vi "UHR-Fleezers Control (host) - 10.0.vi"() -> ()   [LabVIEW 2009] (continued)
              }
            }
          }
        }
        n1053 = node-c288(w4126) -> ()  [unwired: 1 out]
      }
      n1054 = node-c288(w4110) -> ()  [unwired: 1 out]
      n1055 = call "DMR_CloseDevice.vi"("driver handle IN"=w4115) -> ()  [unwired: 1 in, 4 out]
    }
    frame #4 {
      n1056 = call "DMR_Close.vi"() -> ()  [unwired: 1 out]
    }
  }
  n1057 = disable-structure shown="Disabled" {
    disable-tunnel: [w4249 _] -> w213
    disable-tunnel: w14 -> [w4248 _]
    frame #0 {
      n1058 = node-c288() -> (w4251:T22)  [unwired: 4 out]
      n1059 = timed-loop "Rough control of MCL mirror stage (debugging)" {
        tunnel: w4248 -> [w4254]
        tunnel: [w4253] -> w4249
        timing: w4251 -> [_]
        timing-out: [_] -> w4250
        stop <- w4253 stop-if-true
        n1060 = node-c288() -> ()  [unwired: 2 out]
        n1061 = case shown="1" "MCL Mode" {
          tunnel: w4254 -> [_ w4257 w4359]
          frame #0 {
          }
          frame #1 {
            n1062 = node-c288() -> (w4259:T22)  [unwired: 4 out]
            n1063 = timed-loop "Oscillate MCL mirror" {
              timing: w4259 -> [_]
              timing-out: [_] -> w4258
              tunnel: w4257 -> [w4298]
              i -> [w4297]
              stop <- w4260 stop-if-true
              n1064 = node-c288() -> (w4296:i64)  [unwired: 1 out]
              n1065 = Multiply(x="AO1", y=32767.0) -> (x*y=w4292:dbl)
              n1066 = Multiply(x="AO2", y=32767.0) -> (x*y=w4287:dbl)
              n1067 = Divide(x=w4292, y=10.0) -> (x/y=w4293:dbl)
              n1068 = Divide(x=w4287, y=10.0) -> (x/y=w4288:dbl)
              n1069 = To Word Integer(number=w4293) -> (16bit integer=w4285:i16)
              n1070 = To Word Integer(number=w4288) -> (16bit integer=w4284:i16)
              n1071 = Divide(x=w4296, y=i64 1000) -> (x/y=w4267:dbl)
              n1072 = Multiply(x=w4267, y=w4297) -> (x*y=w4278:dbl)
              n1073 = Multiply(x="Osc. freq. (Hz) 2", y=6.283185307179586) -> (x*y=w4279:dbl)
              n1074 = Multiply(x=w4279, y=w4278) -> (x*y=w4277:dbl)
              n1075 = Sine(x=w4277) -> (sin(x)=w4276:dbl)
              n1076 = Multiply(x=w4276, y="Osc. amp. (V)") -> (x*y=w4274:dbl)
              n1077 = Add(x=w4274, y="Osc. center (V)") -> (x+y=w4272:dbl)
              n1078 = Divide(x=w4272, y=10.0) -> (x/y=w4270:dbl)
              n1079 = Multiply(x=w4270, y=32767.0) -> (x*y=w4265:dbl)
              n1080 = Select(t=w4265, s="Scan axis", f=w4285) -> (s? t:f=w4283:dbl)
              n1081 = Select(t=w4284, s="Scan axis", f=w4265) -> (s? t:f=w4282:dbl)
              n1082 = local read "MCL Mode"() -> (w4264:u16)
              n1083 = Not Equal?(x=w4264, y=u16 1) -> (x != y?=w4261:bool)
              n1084 = local read "Stop All"() -> (w4262:bool)
              n1085 = xnode "Read/Write Control"("FPGA VI Reference In"=w4298, "AO1"=w4283, "AO2"=w4282) -> ()  [unwired: 1 in, 2 out]
              n1086 = Compound Arithmetic op=OR(w4262, w4261) -> (w4260:bool)
              n1087 = node-c288() -> ()  [unwired: 2 out]
            }
            n1088 = node-c288(w4258) -> ()  [unwired: 1 out]
          }
          frame #2 {
            n1089 = case shown="True" "Start Scan" {
              tunnel: w4359 -> [_ w4371]
              frame #0 {
              }
              frame #1 {
                n1090 = Subtract(x="End (V)", y="Begin (V)") -> (x-y=w4367:dbl)
                n1091 = Decrement(x="N Points") -> (x-1=w4366:dbl)
                n1092 = Divide(x=w4367, y=w4366) -> (x/y=w4364:dbl)
                n1093 = for {
                  N: "N Points" -> [_]
                  tunnel: "Begin (V)" -> [w4384]
                  tunnel: w4371 -> [w4376]
                  tunnel: [w4375] -> w4370 mode=indexing
                  tunnel: w4364 -> [w4374]
                  tunnel: [w4372] -> w4363 mode=indexing
                  i -> [w4383]
                  n1094 = Multiply(x=w4374, y=w4383) -> (x*y=w4382:dbl)
                  n1095 = Add(x=w4384, y=w4382) -> (x+y=w4379:dbl)
                  n1096 = local read "Scan axis"() -> (w4373:bool)
                  n1097 = local read "AO1"() -> (w4381:dbl)
                  n1098 = local read "AO2"() -> (w4380:dbl)
                  n1099 = Select(t=w4379, s=w4373, f=w4381) -> (s? t:f=w4378:dbl)
                  n1100 = Select(t=w4380, s=w4373, f=w4379) -> (s? t:f=w4377:dbl)
                  n1101 = flat-sequence {
                    tunnel: w4378 -> [w4388]
                    tunnel: w4377 -> [w4387]
                    tunnel: w4376 -> [w4385]
                    tunnel: [w4453] -> w4375
                    tunnel: [w4452] -> w4372
                    frame #0 {
                      w4391 = 10.0 ("y")
                      w4386 = 32767.0 ("y")
                      n1102 = Multiply(x=w4388, y=w4386) -> (x*y=w4394:dbl)
                      n1103 = Multiply(x=w4387, y=w4386) -> (x*y=w4392:dbl)
                      n1104 = Divide(x=w4394, y=w4391) -> (x/y=w4395:dbl)
                      n1105 = Divide(x=w4392, y=w4391) -> (x/y=w4393:dbl)
                      n1106 = To Word Integer(number=w4395) -> (16bit integer=w4389:i16)
                      n1107 = To Word Integer(number=w4393) -> (16bit integer=w4390:i16)
                      n1108 = xnode "Read/Write Control"("FPGA VI Reference In"=w4385, "AO1"=w4389, "AO2"=w4390) -> ()  [unwired: 1 in, 2 out]
                    }
                    frame #1 {
                      n1109 = Wait (ms)(milliseconds to wait="DAQ Delay (ms)") -> ()  [unwired: 1 out]
                    }
                    frame #2 {
                      n1110 = local read "Slow mean"() -> (w4453:dbl)
                      n1111 = local read "Sigma"() -> (w4452:dbl)
                    }
                  }
                }
                n1112 = Bundle("Begin (V)"="Begin (V)", w4364, w4370) -> (→"MCL Scan":cluster{"Begin (V)":dbl, dbl, dbl[]})  [unwired: 1 out]
                n1113 = Bundle("Begin (V)"="Begin (V)", w4364, w4363) -> (→"MCL Scan 2":cluster{"Begin (V)":dbl, dbl, dbl[]})  [unwired: 1 out]
              }
            }
          }
        }
        n1114 = local read "Stop All"() -> (w4253:bool)
        n1115 = node-c288() -> ()  [unwired: 2 out]
      }
      n1116 = node-c288(w4250) -> ()  [unwired: 1 out]
    }
    frame #1 {
    }
  }
  n1117 = timed-loop "Control parameters (event loop)" {
    tunnel: w14 -> [w4460]
    shift-right: [w4459] -> _
    shift-left: errorcluster {"status"=FALSE, "code"=0, "source"=""} ("error out") -> [w4458]
    tunnel: [w4457] -> w211
    timing: w52 -> [_]
    timing-out: [_] -> w51
    tunnel: w22 -> [w4456]
    stop <- w4457 stop-if-true
    n1118 = node-c288() -> ()  [unwired: 2 out]
    n1119 = event shown="[50] \"Set SP to Reading\": Value Change" {
      selector: _ -> [_ _ _ _ _ _ _ _ _ _ _ _ _ _ _ _ _ _ _ _ _ _ _ _ _ _ _ _ _ _ _ _ _ _ _ _ _ _ _ _ _ _ _ _ _ _ _ _ _ _ _ _]
      dyn-events: _ -> [_ _ _ _ _ _ _ _ _ _ _ _ _ _ _ _ _ _ _ _ _ _ _ _ _ _ _ _ _ _ _ _ _ _ _ _ _ _ _ _ _ _ _ _ _ _ _ _ _ _ _ _]
      timeout: _ -> [_ _ _ _ _ _ _ _ _ _ _ _ _ _ _ _ _ _ _ _ _ _ _ _ _ _ _ _ _ _ _ _ _ _ _ _ _ _ _ _ _ _ _ _ _ _ _ _ _ _ _ _]
      tunnel: w4460 -> [w4507 _ _ _ w4643 _ w4738 _ _ _ _ w4804 _ _ w4904 w5042 w5104 w5147 w5297 w5372 w5483 w5576 w5660 w5744 w5828 w5912 w5996 w6089 w6284 w6484 w6577 w6710 _ w6880 w6921 w6968 w7045 w7086 _ w7131 _ _ _ _ w7312 _ w7403 w7443 w7489 w7625 w7673 _]
      tunnel: [w4506 _ _ _ w4633 _ w4737 _ _ w4769 _ w4783 _ _ w4903 w5038 w5101 w5144 w5296 w5370 w5482 w5570 w5654 w5738 w5822 w5906 w5990 w6087 w6283 w6482 w6575 w6708 _ w6878 w6919 w6958 w7043 w7084 _ w7129 _ _ _ _ w7310 _ _ _ _ _ _ _] -> w4459
      tunnel: w4458 -> [w4505 _ _ _ w4642 _ w4736 _ _ w4769 _ w4803 _ _ w4902 w5037 w5100 w5143 w5295 w5371 w5481 w5575 w5659 w5743 w5827 w5911 w5995 w6088 w6282 w6483 w6576 w6709 _ w6879 w6920 w6967 w7044 w7085 _ w7130 _ _ _ _ w7311 _ w7402 w7442 w7488 w7624 w7672 _]
      tunnel: [_ _ _ _ _ _ _ _ _ w4768 _ _ _ _ _ _ _ _ _ _ _ _ _ _ _ _ _ _ _ _ _ _ _ _ _ _ _ _ _ _ _ _ _ _ _ _ _ _ _ _ _ _] -> w4457
      tunnel: [_ _ _ _ _ _ _ "Round T1 X" _ _ _ _ "Load parameters" _ _ _ _ _ _ _ _ _ _ _ _ _ _ _ _ _ _ _ _ _ _ _ _ _ _ _ _ _ _ _ _ _ _ _ _ _ _ _] -> _
      tunnel: [_ _ _ "Adjust Scale\nto Mean" _ _ _ _ _ _ _ _ _ _ _ _ _ _ _ _ _ _ _ _ _ _ _ _ _ _ _ _ _ _ _ _ _ _ _ _ _ _ _ _ _ _ _ _ _ _ "Set SP to Reading" _] -> _
      tunnel: [_ _ _ _ _ _ _ _ "Round T2 X" _ "Delayed Interlace Start" _ _ _ _ _ _ _ _ _ _ _ _ _ _ _ _ _ _ _ _ _ _ _ _ _ _ _ _ _ _ _ _ _ _ _ _ _ _ _ _ _] -> _
      tunnel: [_ "Rescale on Mean" _ _ _ _ _ _ _ _ _ _ _ _ _ _ _ _ _ _ _ _ _ _ _ _ _ _ _ _ _ _ _ _ _ _ _ _ _ _ _ _ _ _ _ _ _ _ _ _ _ _] -> _
      tunnel: w4456 -> [_ _ _ _ _ _ _ _ _ _ _ _ _ _ _ _ _ _ _ _ _ _ _ _ _ _ _ _ _ _ _ _ _ _ _ _ _ _ _ _ _ _ _ w7303 _ _ _ _ _ _ _ _]
      event #0 {
        # "So that if 'Save ave N' is updated, the AOD scanning code updates too."
        n1120 = event-data() -> ()  [unwired: 6 out]
        n1121 = local read "AI Count (ticks)"() -> (w4480:u32)
        n1122 = local read "FPGA Ave."() -> (w4465:dbl)
        n1123 = Boolean To (0,1)(Boolean="Sets to FIFO (Traps)") -> (0, 1=w4495:cluster{"Set 1":i16, "Set 2":i16, "Set 3":i16})
        n1124 = xnode "Read/Write Control"("FPGA VI Reference In"=w4507, "error in"=w4505, "ai count"=w4480, "AI1 Sets to FIFO"="Sets to FIFO (Traps)", "AI Averages"=w4465, "N of AI1 Int Acq Sets"="N Acq Sets (Traps + Fl.)") -> ("error out"=w4506:errorcluster)  [unwired: 1 out]
        n1125 = Cluster To Array(cluster=w4495) -> (array=w4494:i16[])
        n1126 = local read "Scan steps (AOD)"() -> (w4496:u64)
        n1127 = Multiply(x=w4480, y="N Acq Sets (Traps + Fl.)") -> (x*y=w4478:u32)
        n1128 = Divide(x=40000000.0, y=w4480) -> (x/y=w4503:dbl)
        "AI rate (Hz)" <- w4503
        n1129 = Add Array Elements(numeric array=w4494) -> (sum=w4482:i16)
        "Trap Sets" <- w4482
        n1130 = Divide(x=w4503, y=w4465) -> (x/y=w4504:dbl)
        "Ave. Rate (Hz)" <- w4504
        n1131 = Reciprocal(x=w4504) -> (1/x=→"Ave. Period (s)":dbl)
        n1132 = property on="Scan steps (AOD)" class="DigNum (strict)"("Val(Sgnl)"=w4496) -> ()  [unwired: 2 in, 2 out]
        n1133 = Divide(x=w4504, y="N Acq Sets (Traps + Fl.)") -> (x/y=w4500:dbl)
        "Data Rate (Hz)" <- w4500
        n1134 = Reciprocal(x=w4500) -> (1/x=→"Data Period (s)":dbl)
        n1135 = local read "Save ave N"() -> (w4499:dbl)
        n1136 = Divide(x=w4500, y=w4499) -> (x/y=w4498:dbl)
        "Save Data Rate (Hz)" <- w4498
        n1137 = Reciprocal(x=w4498) -> (1/x=→"Save Data Period (s)":dbl)
        n1138 = Multiply(x=w4478, y="# Samples/trap") -> (x*y=w4474:dbl)
        "Counts/DMA" <- w4474
        n1139 = Multiply(x=w4482, y="# Samples/trap") -> (x*y=w4481:dbl)
        "# Samples/channel" <- w4481
        n1140 = Greater?(x=w4465, y=1.0) -> (0:w4469:bool)
        "FPGA Averaging" <- w4469
        n1141 = local read "APD Int. Count"() -> (w4476:u32)
        n1142 = Divide(x=w4481, y=u32 2) -> (x/y=w4487:dbl)
        n1143 = Select(t=w4481, s=w4469, f=w4487) -> (s? t:f=w4492:dbl)
        n1144 = Divide(x=w4474, y=w4476) -> (x/y=w4475:dbl)
        "APD Samples/FIFO Acq." <- w4475
        n1145 = Divide(x=w4474, y=40000000.0) -> (x/y=w4472:dbl)
        "DMA Update Period (s)" <- w4472
        n1146 = Multiply(x=w4492, y=u32 8) -> (x*y=w4468:dbl)
        "Trap AI Elements/DMA read" <- w4468
        n1147 = Divide(x=w4468, y=8.0) -> (x/y=w4466:dbl)
        n1148 = Divide(x=w4468, y=4.0) -> (x/y=w4470:dbl)
        n1149 = Multiply(x=2.0, y=w4475) -> (x*y=→"APD Elements/DMA read":dbl)
        n1150 = Multiply(x=w4465, y=w4466) -> (x*y=w4464:dbl)
        n1151 = Select(t=w4464, s=w4469, f=w4470) -> (s? t:f=→"Trap Pos Elements/DMA read":dbl)
        n1152 = local read "N sets to save"() -> (w4489:u32)
        n1153 = Multiply(x=w4472, y=w4489) -> (x*y=→"Total Time (s)":dbl)
      }
      event #1 {
        n1154 = event-data() -> ()  [unwired: 7 out]
        n1155 = local read "Bead Mean (nm)"() -> (w4612:dbl)
        n1156 = Add(x="Amplitude (nm)", y=w4612) -> (x+y=w4610:dbl)
        n1157 = Subtract(x=w4612, y="Amplitude (nm)") -> (x-y=w4609:dbl)
        n1158 = property on="Bead Separation" class="WFChart (strict)"("YScale.Minimum"=w4609) -> ()  [unwired: 2 in, 2 out]
        n1159 = property on="Bead Separation" class="WFChart (strict)"("YScale.Maximum"=w4610) -> ()  [unwired: 2 in, 2 out]
      }
      event #2 {
        n1160 = event-data() -> ()  [unwired: 7 out]
        n1161 = local read "AI labels"() -> (w4614:string[])
        n1162 = property on="High Res. Display" class="Ring (strict)"("Strings []"=w4614) -> ()  [unwired: 2 in, 2 out]
        n1163 = Build Array (concatenate)(w4614, "none") -> (w4615:string[])
        n1164 = property on="FFT 1 Choice 1" class="Ring (strict)"("Strings []"=w4615) -> ()  [unwired: 2 in, 2 out]
        n1165 = property on="FFT 1 Choice 2" class="Ring (strict)"("Strings []"=w4615) -> ()  [unwired: 2 in, 2 out]
        n1166 = property on="FFT 2 Choice 1" class="Ring (strict)"("Strings []"=w4615) -> ()  [unwired: 2 in, 2 out]
        n1167 = property on="FFT 2 Choice 2" class="Ring (strict)"("Strings []"=w4615) -> ()  [unwired: 2 in, 2 out]
        n1168 = Bundle("APD 1", "APD 2") -> (w4618:cluster{string, string})  [unwired: 1 out]
        n1169 = Cluster To Array(cluster=w4618) -> (array=w4616:string[])
        n1170 = Build Array (concatenate)(w4616, w4615) -> (w4620:string[])
        n1171 = Array Size(array=w4620) -> (size(s)=w4621:i32)
        n1172 = property on="Signals to Plot" class="LstBox (strict)"("Item Names"=w4620) -> ()  [unwired: 2 in, 2 out]
        n1173 = property on="Signals to Plot" class="LstBox (strict)"("Number of Rows"=w4621) -> ()  [unwired: 2 in, 2 out]
        n1174 = property on="All Signals" class="WFChart (strict)"("LegNumRows"=w4621) -> ()  [unwired: 2 in, 2 out]
      }
      event #3 {
        n1175 = event-data() -> ()  [unwired: 7 out]
        n1176 = local read "APD 1 Rate (Hz)"() -> (w4630:dbl)
        n1177 = Multiply(x=1000.0, y="Above (kHz)") -> (x*y=w4628:dbl)
        n1178 = Multiply(x=1000.0, y="Below (kHz)") -> (x*y=w4626:dbl)
        n1179 = Add(x=w4628, y=w4630) -> (x+y=w4623:dbl)
        n1180 = Subtract(x=w4630, y=w4626) -> (x-y=w4624:dbl)
        n1181 = property on="APD Chart" class="WFChart (strict)"("YScale.Minimum"=w4624) -> ()  [unwired: 2 in, 2 out]
        n1182 = property on="APD Chart" class="WFChart (strict)"("YScale.Maximum"=w4623) -> ()  [unwired: 2 in, 2 out]
      }
      event #4 {
        n1183 = event-data() -> ()  [unwired: 7 out]
        n1184 = Negate(x="Phase adj. (AI1)") -> (-x=w4640:i16)
        n1185 = Select(t=w4640, s="- phase (AI1)", f="Phase adj. (AI1)") -> (s? t:f=w4639:i16)
        n1186 = xnode "Read/Write Control"("FPGA VI Reference In"=w4643, "error in"=w4642, "Phase count adjustment"=w4639) -> ("FPGA VI Reference Out"=w4638:T20, "error out"=w4637:errorcluster)
        n1187 = Or(x="- phase (AI1)", y="+ phase (AI1)") -> (x .or. y?=w4634:bool)
        n1188 = xnode "Read/Write Control"("FPGA VI Reference In"=w4638, "error in"=w4637, "+ phase"=w4634) -> ("error out"=w4633:errorcluster)  [unwired: 1 out]
      }
      event #5 {
        w4719 = u32 9868950 ("Color Box")
        n1189 = event-data() -> ("Row"=w4721:i32)  [unwired: 9 out]
        n1190 = property on="All Signals" class="WFChart (strict)"("Active Plot"=w4721) -> (error out=w4732:errorcluster)  [unwired: 2 in, 1 out]
        n1191 = property on="All Signals" class="WFChart (strict)" props=["Plot", "Visible?", "Plot", "Plot Color"](error in=w4732) -> (error out=w4731:errorcluster, "Plot.Visible?"=w4730:bool)  [unwired: 1 in, 2 out]
        n1192 = Select(t=FALSE ("Plot.Visible"), s=w4730, f=TRUE ("Plot.Visible")) -> (s? t:f=w4725:bool)
        n1193 = property on="All Signals" class="WFChart (strict)"(error in=w4731, "Plot.Visible?"=w4725) -> (error out=w4727:errorcluster)  [unwired: 1 in, 1 out]
        n1194 = property on="All Signals" class="WFChart (strict)"(error in=w4727) -> (error out=w4722:errorcluster, "Plot.Plot Color"=w4726:u32)  [unwired: 1 in, 1 out]
        n1195 = property on="Signals to Plot" class="LstBox (strict)"(error in=w4722, "Active Row"=w4721) -> (error out=w4720:errorcluster)  [unwired: 1 in, 1 out]
        n1196 = Select(t=w4726, s=w4725, f=u32 0) -> (s? t:f=w4723:u32)
        n1197 = property on="Signals to Plot" class="LstBox (strict)"(error in=w4720, "CellFontColor"=w4723, "SelColor"=w4719, "CellBG"=w4719, "CellFontSize"=u32 20 ("Active Row:Cell Font:Size"), "CellFontBold"=TRUE ("Active Row:Cell Font:Bold")) -> ()  [unwired: 1 in, 2 out]
      }
      event #6 {
        n1198 = event-data() -> ("CtlRef"=w4735:refnum<vi>)  [unwired: 6 out]
        n1199 = control-ref of="Trap Delta (MHz)"() -> (w4734:refnum<vi>)
        n1200 = Equal?(x=w4734, y=w4735) -> (x = y?=w4733:bool)
        n1201 = case shown="False" "Oscillate Set 1" {
          tunnel: w4738 -> [w4758 _]
          tunnel: [w4757 w4761] -> w4737
          tunnel: w4736 -> [w4756 w4761]
          tunnel: w4733 -> [w4741 _]
          frame #0 {
            n1202 = local read "BD 1 Frequency 2 (MHz)"() -> (w4745:dbl)
            n1203 = local read "BD 1 Frequency 1 (MHz)"() -> (w4743:dbl)
            n1204 = Subtract(x=w4745, y="Trap Delta (MHz)") -> (x-y=w4742:dbl)
            n1205 = Select(t=w4742, s=w4741, f=w4743) -> (s? t:f=w4740:dbl)
            n1206 = local read "Y RF Frequency Limits (MHz)"() -> (w4746:T15)
            n1207 = local read "X RF Frequency Limits (MHz)"() -> (w4747:T15)
            n1208 = local read "BD 1 Frequency 3 (MHz)"() -> (w4759:dbl)
            n1209 = local write "BD 1 Frequency 1 (MHz)"(w4740) -> ()
            n1210 = local read "BD 2 Frequency 1 (MHz)"() -> (w4750:dbl)
            n1211 = local read "BD 2 Frequency 2 (MHz)"() -> (w4749:dbl)
            n1212 = local read "BD 2 Frequency 3 (MHz)"() -> (w4760:dbl)
            n1213 = call "set RF board frequency - interlace.vi"("Board 2 Frequency Limits"=w4746, "Board 1 Frequency Limits"=w4747, "error in"=w4756, "FPGA VI Reference In"=w4758, "Board 2 Frequency 3 (MHz)"=w4760, "Board 1 Frequency 3 (MHz)"=w4759, "Board 2 Frequency 2 (MHz)"=w4749, "Board 2 Frequency 1 (MHz)"=w4750, "Board 1 Frequency 2 (MHz)"=w4745, "Board 1 Frequency 1  (MHz)"=w4740) -> ("error out"=w4757:errorcluster)  [unwired: 1 out]
            n1214 = Subtract(x=w4750, y=w4749) -> (x-y=w4754:dbl)
            n1215 = Subtract(x=w4740, y=w4745) -> (x-y=w4755:dbl)
            n1216 = Square(x=w4754) -> (x^2=w4752:dbl)
            n1217 = Square(x=w4755) -> (x^2=w4753:dbl)
            n1218 = Add(x=w4753, y=w4752) -> (x+y=w4751:dbl)
            n1219 = Square Root(x=w4751) -> (sqrt(x)=w4748:dbl)
            n1220 = local write "Trap Delta (MHz)"(w4748) -> ()
            n1221 = property on="Initial delta (MHz)" class="DigNum (strict)"("Val(Sgnl)"=w4748) -> ()  [unwired: 2 in, 2 out]
          }
          frame #1 {
          }
        }
      }
      event #7 {
        n1222 = event-data() -> ()  [unwired: 7 out]
        n1223 = local read "BD 1 Frequency 1 (MHz)"() -> (w4764:dbl)
        n1224 = Round To Nearest(number=w4764) -> (nearest integer value=w4763:dbl)
        n1225 = property on="BD 1 Frequency 1 (MHz)" class="DigNum (strict)"("Val(Sgnl)"=w4763) -> ()  [unwired: 2 in, 2 out]
      }
      event #8 {
        n1226 = event-data() -> ()  [unwired: 7 out]
        n1227 = local read "BD 1 Frequency 2 (MHz)"() -> (w4766:dbl)
        n1228 = Round To Nearest(number=w4766) -> (nearest integer value=w4765:dbl)
        n1229 = property on="BD 1 Frequency 2 (MHz)" class="DigNum (strict)"("Val(Sgnl)"=w4765) -> ()  [unwired: 2 in, 2 out]
      }
      event #9 {
        n1230 = event-data() -> ()  [unwired: 7 out]
        n1231 = local read "Stop All"() -> (w4768:bool)
      }
      event #10 {
        n1232 = event-data() -> ()  [unwired: 7 out]
        n1233 = flat-sequence {
          frame #0 {
            n1234 = Multiply(x="Delay to Interlace (s)", y=1000.0) -> (x*y=w4771:dbl)
            n1235 = Wait (ms)(milliseconds to wait=w4771) -> ()  [unwired: 1 out]
          }
          frame #1 {
            n1236 = property on="Green laser mode" class="RadioBtnsControl (strict)"("Val(Sgnl)"=enum32{"Laser ON", "Laser OFF", "Interlace"}."Interlace" ("Value (Signaling)")) -> ()  [unwired: 2 in, 2 out]
          }
        }
      }
      event #11 {
        w4795 = i16 1 ("f")
        n1237 = event-data() -> ()  [unwired: 7 out]
        n1238 = local write "Trap 1 (ON/OFF)"("Trap 1 ON") -> ()
        n1239 = local write "Trap 2 (ON/OFF)"("Trap 2 ON") -> ()
        n1240 = Boolean To (0,1)(Boolean="Trap 3 ON") -> (0, 1=w4796:i16)
        n1241 = Boolean To (0,1)(Boolean="Trap 1 ON") -> (0, 1=w4797:i16)
        n1242 = Boolean To (0,1)(Boolean="Trap 2 ON") -> (0, 1=w4798:i16)
        n1243 = Select(t=w4798, s="Trap ON/OFF X or Y Amp?", f=w4795) -> (s? t:f=w4793:i16)
        n1244 = Select(t=w4797, s="Trap ON/OFF X or Y Amp?", f=w4795) -> (s? t:f=w4794:i16)
        n1245 = Select(t=w4796, s="Trap ON/OFF X or Y Amp?", f=w4795) -> (s? t:f=w4792:i16)
        n1246 = Select(t=w4795, s="Trap ON/OFF X or Y Amp?", f=w4798) -> (s? t:f=w4790:i16)
        n1247 = Select(t=w4795, s="Trap ON/OFF X or Y Amp?", f=w4797) -> (s? t:f=w4791:i16)
        n1248 = Select(t=w4795, s="Trap ON/OFF X or Y Amp?", f=w4796) -> (s? t:f=w4789:i16)
        n1249 = And(x="All FB On/Off", y="Feedback On/Off") -> (x .and. y?=w4787:cluster{"Set 1":bool, "Set 2":bool})
        n1250 = local read "BD 1 Amplitude 1 (%)"() -> (w4807:dbl)
        n1251 = local read "BD 1 Amplitude 2 (%)"() -> (w4806:dbl)
        n1252 = local read "BD 1 Amplitude 3 (%)"() -> (w4805:dbl)
        n1253 = Unbundle By Name(w4787) -> ("Set 1"=w4782:bool, "Set 2"=w4779:bool)
        n1254 = local read "Y RF Amplitude Limits (%)"() -> (w4775:T15)
        n1255 = local read "X RF Amplitude Limits (%)"() -> (w4776:T15)
        n1256 = local read "BD 2 Amplitude 1 (%)"() -> (w4808:dbl)
        n1257 = local read "BD 2 Amplitude 2 (%)"() -> (w4809:dbl)
        n1258 = local read "BD 2 Amplitude 3 (%)"() -> (w4810:dbl)
        n1259 = And(x="Trap 2 ON", y=w4779) -> (x .and. y?=w4777:bool)
        n1260 = And(x="Trap 1 ON", y=w4782) -> (x .and. y?=w4780:bool)
        n1261 = Multiply(x=w4794, y=w4807) -> (x*y=w4802:dbl)
        n1262 = Multiply(x=w4806, y=w4793) -> (x*y=w4800:dbl)
        n1263 = Multiply(x=w4805, y=w4792) -> (x*y=w4801:dbl)
        n1264 = Multiply(x=w4808, y=w4791) -> (x*y=w4811:dbl)
        n1265 = Multiply(x=w4809, y=w4790) -> (x*y=w4812:dbl)
        n1266 = Multiply(x=w4810, y=w4789) -> (x*y=w4813:dbl)
        n1267 = call "set RF board amplitude - interlace.vi"("Board 2 Amplitude Limits"=w4775, "Board 1 Amplitude Limits"=w4776, "error in"=w4803, "FPGA VI Reference In"=w4804, "Board 2 Amplitude 3 (%)"=w4813, "Board 1 Amplitude 3 (%)"=w4801, "Board 2 Amplitude 2 (%)"=w4812, "Board 2 Amplitude 1 (%)"=w4811, "Board 1 Amplitude 2 (%)"=w4800, "Board 1 Amplitude 1 (%)"=w4802) -> ("error out"=w4784:errorcluster, "FPGA VI Reference Out"=w4785:T20)
        n1268 = xnode "Read/Write Control"("FPGA VI Reference In"=w4785, "error in"=w4784, "FB On/Off Set 1"=w4780, "FB On/Off Set 2"=w4777) -> ("error out"=w4783:errorcluster)  [unwired: 1 out]
      }
      event #12 {
        n1269 = event-data() -> ()  [unwired: 7 out]
        n1270 = property on="Saved AOD Raster Scan Parameter Sets" class="Arr (strict)"() -> ("Index Values"=w4880:u32[])  [unwired: 2 in, 2 out]
        n1271 = Index Array(array=w4880, index=0) -> (element=w4877:u32)
        n1272 = Index Array(array="Saved AOD Raster Scan Parameter Sets", index=w4877) -> (element=w4876:T43)
        n1273 = Unbundle By Name(w4876) -> ("Scan Range AOD (nm) 2"=w4875:dbl, "Step Size AOD (nm) 2"=w4874:dbl, "Scan Speed AOD (nm/s) 2"=w4873:dbl, "Number of scans (AOD) 2"=w4872:u16)
        n1274 = flat-sequence {
          tunnel: w4875 -> [w4884]
          tunnel: w4874 -> [w4883]
          tunnel: w4873 -> [w4882]
          tunnel: w4872 -> [w4885]
          frame #0 {
            n1275 = local write "Scan Speed (nm/s)"(w4882) -> ()
            n1276 = local write "Scan Range (nm)"(w4884) -> ()
            n1277 = local write "Step Size (nm)"(w4883) -> ()
          }
          frame #1 {
            n1278 = property on="Number of F/B Scans (AOD)" class="DigNum (strict)"("Val(Sgnl)"=w4885) -> ()  [unwired: 2 in, 2 out]
          }
        }
      }
      event #13 {
        n1279 = event-data() -> ()  [unwired: 7 out]
        n1280 = property on="Trap 2 ON" class="Bool (strict)"("Val(Sgnl)"="Trap 2 (ON/OFF)") -> ()  [unwired: 2 in, 2 out]
        n1281 = property on="Trap 1 ON" class="Bool (strict)"("Val(Sgnl)"="Trap 1 (ON/OFF)") -> ()  [unwired: 2 in, 2 out]
      }
      event #14 {
        n1282 = event-data() -> ()  [unwired: 7 out]
        n1283 = local read "DIO count 3 (ticks)"() -> (w4898:u32)
        n1284 = local read "DIO count 1 (ticks)"() -> (w4900:u32)
        n1285 = local read "DIO count 2 (ticks)"() -> (w4899:u32)
        n1286 = To Unsigned Byte Integer(number="Not-Interlacing Set") -> (unsigned 8bit integer=w4889:u8)
        n1287 = Add(x=w4889, y=u8 1) -> (x+y=w4893:u8)
        n1288 = xnode "Read/Write Control"("FPGA VI Reference In"=w4904, "error in"=w4902, "DIO count 1 (ticks)"=w4900, "DIO count 2 (ticks)"=w4899, "DIO count 3 (ticks)"=w4898, "Interlace ON/OFF"="Interlace", "Number Interlace Cycles"="Number Interlace Sets", "Interlace Off Parameters"=w4893) -> ("error out"=w4903:errorcluster)  [unwired: 1 out]
        n1289 = Build Array(w4900, w4899, w4898) -> (w4891:u32[])
        n1290 = Split 1D Array(array=w4891, index="Number Interlace Sets") -> (first subarray=w4901:u32[])  [unwired: 1 out]
        n1291 = Index Array(array=w4891, index=w4889) -> (element=w4890:u32)
        n1292 = Add Array Elements(numeric array=w4901) -> (sum=w4895:u32)
        n1293 = Select(t=w4895, s="Interlace", f=w4890) -> (s? t:f=→"Total Counts (ticks)":u32)
      }
      event #15 {
        n1294 = event-data() -> ()  [unwired: 7 out]
        n1295 = Unbundle By Name("Reset Feedback") -> ("Set 1"=w5040:bool, "Set 2"=w5039:bool)
        n1296 = xnode "Read/Write Control"("FPGA VI Reference In"=w5042, "error in"=w5037, "FB Reset Set 1"=w5040, "FB Reset Set 2"=w5039) -> ("error out"=w5038:errorcluster)  [unwired: 1 out]
      }
      event #16 {
        n1297 = event-data() -> ()  [unwired: 7 out]
        n1298 = Unbundle By Name("PID Gains") -> ("Set 1"=w5103:T13, "Set 2"=w5102:T13)
        n1299 = xnode "Read/Write Control"("FPGA VI Reference In"=w5104, "error in"=w5100, "FB Gains Set 1"=w5103, "FB Gains Set 2"=w5102) -> ("error out"=w5101:errorcluster)  [unwired: 1 out]
      }
      event #17 {
        n1300 = event-data() -> ()  [unwired: 7 out]
        n1301 = xnode "Read/Write Control"("FPGA VI Reference In"=w5147, "error in"=w5143) -> ("FPGA VI Reference Out"=w5146:T20, "error out"=w5145:errorcluster, "AI2 Y Sum Set 1"=w5154:i16, "AI2 Y Sum Set 2"=w5153:i16)
        n1302 = Cluster To Array(cluster="AI2 to Setpoint") -> (array=w5157:bool[])
        n1303 = local read "AI2 (V)"() -> (w5155:cluster{"Set 1":dbl, "Set 2":dbl})
        n1304 = Or Array Elements(Boolean array=w5157) -> (logical OR=w5158:bool)
        n1305 = Bundle By Name(cluster=w5155, "Set 1"=w5154, "Set 2"=w5153) -> (w5152:cluster{"Set 1":dbl, "Set 2":dbl})
        n1306 = Divide(x=w5152, y=3276.7) -> (x/y=w5151:cluster{"Set 1":dbl, "Set 2":dbl})
        "AI2 (V)" <- w5151
        n1307 = case shown="True" w5158 {
          tunnel: [w5220 w5237] -> w5150
          tunnel: "AI2 to Setpoint" -> [_ w5233]
          tunnel: "Setpoints (V)" -> [w5221 w5236]
          tunnel: w5151 -> [_ w5230]
          frame #0 {
            n1308 = Multiply(x=3276.7, y=w5221) -> (x*y=w5222:cluster{"Set 1":dbl, "Set 2":dbl})
            n1309 = To Word Integer(number=w5222) -> (16bit integer=w5220:cluster{"Set 1":i16, "Set 2":i16})
          }
          frame #1 {
            n1310 = Unbundle By Name(w5230) -> ("Set 1"=w5229:dbl, "Set 2"=w5228:dbl)
            n1311 = Unbundle By Name(w5236) -> ("Set 1"=w5235:dbl, "Set 2"=w5234:dbl)
            n1312 = Unbundle By Name(w5233) -> ("Set 1"=w5232:bool, "Set 2"=w5231:bool)
            n1313 = Select(t=w5229, s=w5232, f=w5235) -> (s? t:f=w5227:dbl)
            n1314 = Select(t=w5228, s=w5231, f=w5234) -> (s? t:f=w5226:dbl)
            n1315 = Bundle By Name(cluster=w5236, "Set 1"=w5227, "Set 2"=w5226) -> (w5224:cluster{"Set 1":dbl, "Set 2":dbl})
            n1316 = Multiply(x=3276.7, y=w5224) -> (x*y=w5225:cluster{"Set 1":dbl, "Set 2":dbl})
            n1317 = local write "Setpoints (V)"(w5224) -> ()
            n1318 = To Word Integer(number=w5225) -> (16bit integer=w5237:cluster{"Set 1":i16, "Set 2":i16})
          }
        }
        n1319 = Unbundle By Name(w5150) -> ("Set 1"=w5149:i16, "Set 2"=w5148:i16)
        n1320 = xnode "Read/Write Control"("FPGA VI Reference In"=w5146, "error in"=w5145, "FB Setpoint Set 1"=w5149, "FB Setpoint Set 2"=w5148) -> ("error out"=w5144:errorcluster)  [unwired: 1 out]
      }
      event #18 {
        n1321 = event-data() -> ()  [unwired: 7 out]
        n1322 = xnode "Read/Write Control"("FPGA VI Reference In"=w5297, "error in"=w5295, "Invert GI"="Invert GI", "Invert GI 2"="Invert GI") -> ("error out"=w5296:errorcluster)  [unwired: 1 out]
      }
      event #19 {
        n1323 = event-data() -> ()  [unwired: 7 out]
        n1324 = local read "Green FB Setpoint (mV)"() -> (w5361:dbl)
        n1325 = local read "Current When FB OFF (%)"() -> (w5364:dbl)
        n1326 = Multiply(x=w5361, y=3.2767) -> (x*y=w5360:dbl)
        n1327 = Multiply(x=w5364, y=655.35) -> (x*y=w5365:dbl)
        n1328 = To Unsigned Word Integer(number=w5365) -> (unsigned 16bit integer=w5363:u16)
        n1329 = local read "Green int current ON count adj"() -> (w5368:u32)
        n1330 = local read "Green FB Gains"() -> (w5367:T13)
        n1331 = local read "Green Laser ON/Interlacing"() -> (w5358:bool)
        n1332 = local read "Green laser mode"() -> (w5357:enum32{"Laser ON", "Laser OFF", "Interlace"})
        n1333 = local read "Green FB On/Off"() -> (w5369:bool)
        n1334 = Equal?(x=w5357, y=enum32{"Laser ON", "Laser OFF", "Interlace"}."Interlace") -> (x = y?=w5355:bool)
        n1335 = Compound Arithmetic op=AND(w5355, w5369, w5358) -> (w5359:bool)
        n1336 = xnode "Read/Write Control"("FPGA VI Reference In"=w5372, "error in"=w5371, "Green FB Setpoint"=w5360, "Green FB On/Off"=w5359, "Current Out"=w5363, "Green int current ON count adj"=w5368, "Green FB Gains"=w5367) -> ("error out"=w5370:errorcluster)  [unwired: 1 out]
      }
      event #20 {
        n1337 = event-data() -> ()  [unwired: 7 out]
        n1338 = case shown="True" "Green Laser ON/Interlacing" {
          tunnel: "Green laser mode" -> [_ w5490]
          tunnel: [enum32{"Laser ON", "Laser OFF", "Interlace"}."Laser OFF" ("Green laser mode") w5490] -> w5478
          tunnel: [FALSE w5486] -> w5477
          frame #0 {
          }
          frame #1 {
            n1339 = local read "Green FB On/Off"() -> (w5487:bool)
            n1340 = Equal?(x=w5490, y=enum32{"Laser ON", "Laser OFF", "Interlace"}."Interlace") -> (x = y?=w5488:bool)
            n1341 = And(x=w5488, y=w5487) -> (x .and. y?=w5486:bool)
          }
        }
        n1342 = xnode "Read/Write Control"("FPGA VI Reference In"=w5483, "error in"=w5481, "Operating Mode"=w5478, "Operating Mode 2"=w5478, "Green FB On/Off"=w5477) -> ("error out"=w5482:errorcluster)  [unwired: 1 out]
      }
      event #21 {
        n1343 = event-data() -> ()  [unwired: 7 out]
        n1344 = local read "Phase Adj. (APD 1 Gate)"() -> (w5566:i16)
        n1345 = Negate(x=w5566) -> (-x=w5574:i16)
        n1346 = Select(t=w5574, s="- phase (APD 1 Gate)", f=w5566) -> (s? t:f=w5573:i16)
        n1347 = Or(x="- phase (APD 1 Gate)", y="+ phase (APD 1 Gate)") -> (x .or. y?=w5569:bool)
        n1348 = xnode "Read/Write Control"("FPGA VI Reference In"=w5576, "error in"=w5575, "Phase count adjustment (APD 1 Gate)"=w5573) -> ("FPGA VI Reference Out"=w5571:T20, "error out"=w5572:errorcluster)
        n1349 = xnode "Read/Write Control"("FPGA VI Reference In"=w5571, "error in"=w5572, "+ phase (APD 1 Gate)"=w5569) -> ("error out"=w5570:errorcluster)  [unwired: 1 out]
      }
      event #22 {
        n1350 = event-data() -> ()  [unwired: 7 out]
        n1351 = local read "Phase Adj. (APD 2 Gate)"() -> (w5650:i16)
        n1352 = Negate(x=w5650) -> (-x=w5658:i16)
        n1353 = Select(t=w5658, s="- phase (APD 2 Gate)", f=w5650) -> (s? t:f=w5657:i16)
        n1354 = Or(x="- phase (APD 2 Gate)", y="+ phase (APD 2 Gate)") -> (x .or. y?=w5653:bool)
        n1355 = xnode "Read/Write Control"("FPGA VI Reference In"=w5660, "error in"=w5659, "Phase count adjustment (APD 2 Gate)"=w5657) -> ("FPGA VI Reference Out"=w5655:T20, "error out"=w5656:errorcluster)
        n1356 = xnode "Read/Write Control"("FPGA VI Reference In"=w5655, "error in"=w5656, "+ phase (APD 2 Gate)"=w5653) -> ("error out"=w5654:errorcluster)  [unwired: 1 out]
      }
      event #23 {
        n1357 = event-data() -> ()  [unwired: 7 out]
        n1358 = local read "Phase Adj. (APD Acq)"() -> (w5736:i16)
        n1359 = Negate(x=w5736) -> (-x=w5742:i16)
        n1360 = Select(t=w5742, s="+ phase (APD Acq)", f=w5736) -> (s? t:f=w5741:i16)
        n1361 = Or(x="+ phase (APD Acq)", y="- phase (APD Acq)") -> (x .or. y?=w5737:bool)
        n1362 = xnode "Read/Write Control"("FPGA VI Reference In"=w5744, "error in"=w5743, "Phase Count Adjustment (APD Acq)"=w5741) -> ("FPGA VI Reference Out"=w5739:T20, "error out"=w5740:errorcluster)
        n1363 = xnode "Read/Write Control"("FPGA VI Reference In"=w5739, "error in"=w5740, "+ phase (APD Acq)"=w5737) -> ("error out"=w5738:errorcluster)  [unwired: 1 out]
      }
      event #24 {
        n1364 = event-data() -> ()  [unwired: 7 out]
        n1365 = Negate(x="Phase adj. (GI)") -> (-x=w5826:i16)
        n1366 = Select(t=w5826, s="+ phase (GI)", f="Phase adj. (GI)") -> (s? t:f=w5825:i16)
        n1367 = Or(x="+ phase (GI)", y="- phase (GI)") -> (x .or. y?=w5821:bool)
        n1368 = xnode "Read/Write Control"("FPGA VI Reference In"=w5828, "error in"=w5827, "Phase count adjustment (GI)"=w5825) -> ("FPGA VI Reference Out"=w5823:T20, "error out"=w5824:errorcluster)
        n1369 = xnode "Read/Write Control"("FPGA VI Reference In"=w5823, "error in"=w5824, "+ phase (GI)"=w5821) -> ("error out"=w5822:errorcluster)  [unwired: 1 out]
      }
      event #25 {
        n1370 = event-data() -> ()  [unwired: 7 out]
        n1371 = Negate(x="Phase adj. (GI) 2") -> (-x=w5910:i16)
        n1372 = Select(t=w5910, s="+ phase (GI) 2", f="Phase adj. (GI) 2") -> (s? t:f=w5909:i16)
        n1373 = Or(x="+ phase (GI) 2", y="- phase (GI) 2") -> (x .or. y?=w5905:bool)
        n1374 = xnode "Read/Write Control"("FPGA VI Reference In"=w5912, "error in"=w5911, "Phase count adjustment (GI) 2"=w5909) -> ("FPGA VI Reference Out"=w5907:T20, "error out"=w5908:errorcluster)
        n1375 = xnode "Read/Write Control"("FPGA VI Reference In"=w5907, "error in"=w5908, "+ phase (GI) 2"=w5905) -> ("error out"=w5906:errorcluster)  [unwired: 1 out]
      }
      event #26 {
        n1376 = event-data() -> ()  [unwired: 7 out]
        n1377 = Negate(x="Phase adj. (Green FB)") -> (-x=w5994:i16)
        n1378 = Select(t=w5994, s="+ phase (Green FB)", f="Phase adj. (Green FB)") -> (s? t:f=w5993:i16)
        n1379 = Or(x="+ phase (Green FB)", y="- phase (Green FB)") -> (x .or. y?=w5989:bool)
        n1380 = xnode "Read/Write Control"("FPGA VI Reference In"=w5996, "error in"=w5995, "Phase count adjustment (Green FB)"=w5993) -> ("FPGA VI Reference Out"=w5991:T20, "error out"=w5992:errorcluster)
        n1381 = xnode "Read/Write Control"("FPGA VI Reference In"=w5991, "error in"=w5992, "+ phase (Green FB)"=w5989) -> ("error out"=w5990:errorcluster)  [unwired: 1 out]
      }
      event #27 {
        n1382 = event-data() -> ()  [unwired: 7 out]
        n1383 = local read "APD Integration Time (s)"() -> (w6070:dbl)
        n1384 = local read "APD Gate ON Count"() -> (w6085:u32)
        n1385 = local read "APD Gate OFF Count"() -> (w6084:u32)
        n1386 = local read "Invert APD Gate"() -> (w6086:bool)
        n1387 = local read "APD Gate"() -> (w6083:enum32{"ON", "OFF", "Interlace"})
        n1388 = Multiply(x=w6070, y=40000000.0) -> (x*y=w6081:dbl)
        n1389 = Reciprocal(x=w6070) -> (1/x=→"APD Acq Rate (Hz)":dbl)
        n1390 = To Unsigned Long Integer(number=w6081) -> (unsigned 32bit integer=w6080:u32)
        n1391 = local read "DMA Update Period (s)"() -> (w6071:dbl)
        n1392 = Divide(x=w6071, y=w6070) -> (x/y=w6074:dbl)
        n1393 = local read "APD 1 AO offset"() -> (w6076:i16)
        n1394 = local read "APD 1 AO Mult."() -> (w6078:i16)
        n1395 = local read "APD 2 AO Mult."() -> (w6077:i16)
        n1396 = local read "APD 2 AO offset"() -> (w6075:i16)
        n1397 = Multiply(x=2.0, y=w6074) -> (x*y=w6073:dbl)
        n1398 = local write "APD Samples/FIFO Acq."(w6074) -> ()
        n1399 = local write "APD Elements/DMA read"(w6073) -> ()
        n1400 = xnode "Read/Write Control"("FPGA VI Reference In"=w6089, "error in"=w6088, "Invert APD Gate"=w6086, "APD Gate ON Count"=w6085, "APD Gate OFF Count"=w6084, "APD Acq Rate Count"=w6080, "APD Gate Operating Mode"=w6083, "APD 1 AO scale factor"=w6078, "APD 2 AO scale factor"=w6077, "APD 1 AO offset"=w6076, "APD 2 AO offset"=w6075) -> ("error out"=w6087:errorcluster)  [unwired: 1 out]
      }
      event #28 {
        n1401 = event-data() -> ()  [unwired: 7 out]
        n1402 = xnode "Read/Write Control"("FPGA VI Reference In"=w6284, "error in"=w6282, "Green interlace ON count"="GI Frequency, ON count", "Green interlace OFF count"="GI Frequency, OFF count", "Green interlace ON count 2"="GI Frequency, ON count", "Green interlace OFF count 2"="GI Frequency, OFF count", "Green FB Count"="Green FB Count") -> ("error out"=w6283:errorcluster)  [unwired: 1 out]
      }
      event #29 {
        w6452 = 123.0  # AOM cal (nm/MHz)
        n1403 = event-data() -> ()  [unwired: 7 out]
        n1404 = local read "BD 1 Frequency 1 (MHz)"() -> (w6435:dbl)
        n1405 = local read "AOM X Cal (nm/MHz)"() -> (w6427:dbl)
        n1406 = local read "X RF Frequency Limits (MHz)"() -> (w6439:T15)
        n1407 = local read "Y RF Frequency Limits (MHz)"() -> (w6436:T15)
        n1408 = local read "BD 2 Frequency 1 (MHz)"() -> (w6441:dbl)
        n1409 = Negate(x="Scan Range (nm)") -> (-x=w6404:dbl)
        n1410 = Divide(x=w6404, y=w6427) -> (x/y=w6408:dbl)
        n1411 = Select(t=w6439, s="Scan BD", f=w6436) -> (s? t:f=w6438:T15)
        n1412 = Select(t=w6435, s="Scan BD", f=w6441) -> (s? t:f=w6440:dbl)
        n1413 = Unbundle By Name(w6438) -> ("Maximum"=w6447:dbl, "Minimum"=w6446:dbl)
        n1414 = Add(x=w6408, y=w6440) -> (x+y=w6444:dbl)
        n1415 = Divide(x=w6404, y="Step Size (nm)") -> (x/y=w6424:dbl)
        n1416 = Divide(x="Step Size (nm)", y=w6427) -> (x/y=w6433:dbl)
        n1417 = Absolute Value(x=w6424) -> (abs(x)=w6407:dbl)
        n1418 = Sign(1:w6404) -> (0:w6405:dbl)
        n1419 = In Range and Coerce(upper limit=w6447, x=w6444, lower limit=w6446) -> (coerced(x)=w6443:dbl, In Range?=w6445:bool)
        n1420 = To Unsigned Quad Integer(1:w6407) -> (0:w6423:u64)
        "Scan steps (AOD)" <- w6423
        n1421 = call "IR AOM freq to word.vi"("Frequency In (MHz)"=w6433) -> ("Frequency Word Out (double)"=w6430:dbl)
        n1422 = Multiply(x=w6405, y=w6430) -> (x*y=w6406:dbl)
        n1423 = Subtract(x=w6444, y=w6443) -> (x-y=w6442:dbl)
        n1424 = To Quad Integer(1:w6406) -> (0:w6429:i64)
        "Incr. int (AOD)" <- w6429
        n1425 = Subtract(x=w6408, y=w6442) -> (x-y=w6428:dbl)
        "Scan Range (MHz)" <- w6428
        n1426 = Select(t=w6408, s=w6445, f=w6428) -> (s? t:f=w6448:dbl)
        n1427 = Multiply(x=w6428, y=w6427) -> (x*y=w6426:dbl)
        n1428 = Decrement(x=w6423) -> (x-1=w6476:u64)
        n1429 = Negate(x=w6426) -> (-x=w6422:dbl)
        n1430 = local write "Scan Range (nm)"(w6422) -> ()
        n1431 = Divide(x=w6448, y=w6476) -> (x/y=w6432:dbl)
        "Scan Increment (MHz)" <- w6432
        n1432 = call "IR AOM freq to word.vi"("Frequency In (MHz)"=w6432) -> ("Frequency Word Out (double)"=w6431:dbl)
        n1433 = Divide(x="Step Size (nm)", y="Scan Speed (nm/s)") -> (x/y=w6419:dbl)
        n1434 = To Quad Integer(1:w6431) -> ()  [unwired: 1 out]
        n1435 = local read "Number Interlace Sets"() -> (w6402:u8)
        n1436 = local read "AI Count (ticks)"() -> (w6403:u32)
        n1437 = local read "Total Counts (ticks)"() -> (w6401:u32)
        n1438 = local read "# Samples/trap"() -> (w6434:dbl)
        n1439 = Multiply(x=w6403, y=w6402) -> (x*y=w6400:u32)
        n1440 = Divide(x=w6401, y=w6400) -> (x/y=w6399:dbl)
        n1441 = Select(t=w6435, s="Scan BD", f=w6441) -> (s? t:f=w6473:dbl)
        "Initial freq. (MHz)" <- w6473
        n1442 = Add(x=w6448, y=w6473) -> (x+y=→"Final freq. (MHz)":dbl)
        n1443 = Divide(x=w6401, y=40000000.0) -> (x/y=w6418:dbl)
        n1444 = Divide(x=w6419, y=w6418) -> (x/y=w6417:dbl)
        n1445 = To Unsigned Quad Integer(1:w6417) -> (0:w6416:u64)
        "Cycles/step (AOD)" <- w6416
        n1446 = xnode "Read/Write Control"("FPGA VI Reference In"=w6484, "error in"=w6483, "Scan steps"=w6423, "Number of scans"="Number of F/B Scans (AOD)", "Cycles per step"=w6416, "Scan freq.  increment"=w6429, "Scan BD"="Scan BD") -> ("error out"=w6482:errorcluster)  [unwired: 1 out]
        n1447 = Multiply(x=w6423, y=w6416) -> (x*y=w6477:u64)
        n1448 = Multiply(x=w6477, y=u64 2) -> (x*y=w6398:u64)
        n1449 = Multiply(x=w6399, y=w6398) -> (x*y=w6397:dbl)
        "Data points/scan (f/b)" <- w6397
        n1450 = Multiply(x=w6397, y="Number of F/B Scans (AOD)") -> (x*y=w6480:dbl)
        "Data points/scans" <- w6480
        n1451 = Divide(x=w6480, y=w6434) -> (x/y=→"N sets should be saved":dbl)
        n1452 = Multiply(x=w6477, y=w6418) -> (x*y=w6415:dbl)
        "Time/Scan (s) (AOD)" <- w6415
        n1453 = Select(t=w6448, s="Scan BD", f=0.0) -> (s? t:f=w6474:dbl)
        n1454 = Select(t=0.0, s="Scan BD", f=w6448) -> (s? t:f=w6470:dbl)
        n1455 = local read "BD 2 Frequency 2 (MHz)"() -> (w6466:dbl)
        n1456 = local read "BD 1 Frequency 2 (MHz)"() -> (w6469:dbl)
        n1457 = Add(x=w6470, y=w6441) -> (x+y=w6467:dbl)
        n1458 = Add(x=w6435, y=w6474) -> (x+y=w6468:dbl)
        n1459 = Multiply(x=w6415, y=2.0) -> (x*y=w6414:dbl)
        n1460 = Multiply(x=w6414, y="Number of F/B Scans (AOD)") -> (x*y=w6411:dbl)
        n1461 = Divide(x=w6411, y=60.0) -> (x/y=→"Time to Finish All (min)":dbl)
        n1462 = Add(x="Trap 2 Bead Size (nm)", y="Trap 1 Bead Size (nm)") -> (x+y=w6456:dbl)
        n1463 = Divide(x=w6456, y=2.0) -> (x/y=w6450:dbl)
        n1464 = Subtract(x=w6467, y=w6466) -> (x-y=w6464:dbl)
        n1465 = Subtract(x=w6468, y=w6469) -> (x-y=w6465:dbl)
        n1466 = local read "Initial delta (MHz)"() -> (w6453:dbl)
        n1467 = Square(x=w6464) -> (x^2=w6463:dbl)
        n1468 = Square(x=w6465) -> (x^2=w6462:dbl)
        n1469 = Add(x=w6462, y=w6463) -> (x+y=w6461:dbl)
        n1470 = Square Root(x=w6461) -> (sqrt(x)=w6460:dbl)
        "Final delta (MHz)" <- w6460
        n1471 = Multiply(x=w6452, y=w6460) -> (x*y=w6459:dbl)
        n1472 = Multiply(x=w6453, y=w6452) -> (x*y=w6451:dbl)
        n1473 = Subtract(x=w6451, y=w6450) -> (x-y=→"Initial sep (nm)":dbl)
        n1474 = Subtract(x=w6459, y=w6450) -> (x-y=→"Final sep (nm)":dbl)
      }
      event #30 {
        n1475 = event-data() -> ()  [unwired: 7 out]
        n1476 = local read "Freq or Amp switch first"() -> (w6571:bool)
        n1477 = local read "Amp switch delay"() -> (w6572:u16)
        n1478 = local read "Freq switch delay"() -> (w6574:u16)
        n1479 = local read "Swap F1 and F2"() -> (w6573:bool)
        n1480 = xnode "Read/Write Control"("FPGA VI Reference In"=w6577, "error in"=w6576, "Freq switch delay"=w6574, "Swap F1 and F2"=w6573, "Amp switch delay"=w6572, "Freq or Amp switch first"=w6571) -> ("error out"=w6575:errorcluster)  [unwired: 1 out]
      }
      event #31 {
        w6674 = 32767.0 ("y")
        n1481 = event-data() -> ()  [unwired: 7 out]
        n1482 = Select(t="Scan lines (y)", s="2D or 1D Scan", f="Number of scans (MCL)") -> (s? t:f=w6679:u64)
        n1483 = Decrement(x="Scan steps (MCL)") -> (x-1=w6695:u64)
        n1484 = Divide(x="Scan Range (V)\n(of steps)", y=w6695) -> (x/y=w6694:dbl)
        "Desired Scan Incr (V)" <- w6694
        n1485 = local read "APD Integration Time (s)"() -> (w6687:dbl)
        n1486 = Multiply(x=w6694, y=w6674) -> (x*y=w6703:dbl)
        n1487 = Divide(x=w6703, y=10.0) -> (x/y=w6693:dbl)
        "Desired incr (int)" <- w6693
        n1488 = local read "Update Count (MCL)"() -> (w6699:u32)
        n1489 = Round Toward -Infinity(1:w6693) -> (0:w6702:dbl)
        n1490 = To Word Integer(number=w6702) -> (16bit integer=w6677:i16)
        "Actual Incr. int (MCL)" <- w6677
        n1491 = Multiply(x=w6687, y=40000000.0) -> (x*y=w6700:dbl)
        n1492 = Divide(x=w6700, y=w6699) -> (x/y=w6698:dbl)
        n1493 = Multiply(x=i16 10, y=w6677) -> (x*y=w6675:i16)
        n1494 = Multiply(x="N APD Samp/step", y=w6698) -> (x*y=w6697:dbl)
        "Cycles/step (MCL)" <- w6697
        n1495 = Divide(x=w6675, y=w6674) -> (x/y=→"Actual MCL Inc (V)":dbl)
        n1496 = Multiply(x="N APD Samp/step", y="Scan steps (MCL)") -> (x*y=w6689:dbl)
        n1497 = local read "APD Samples/FIFO Acq."() -> (w6686:dbl)
        n1498 = Multiply(x=w6689, y=u64 2) -> (x*y=w6688:dbl)
        "Data points/scan (f+b)" <- w6688
        n1499 = Multiply(x=w6688, y=w6679) -> (x*y=w6706:dbl)
        "Data points/scans (MCL)" <- w6706
        n1500 = Multiply(x=w6687, y=w6688) -> (x*y=w6680:dbl)
        "Time/f+b scan (s) (MCL)" <- w6680
        n1501 = Divide(x=w6706, y=w6686) -> (x/y=→"N sets should be saved (MCL)":dbl)
        n1502 = Multiply(x=w6680, y=w6679) -> (x*y=→"Total Time (s)":dbl)
        n1503 = Not(x="Fast Scan Dir") -> (.not. x?=w6684:bool)
        n1504 = xnode "Read/Write Control"("FPGA VI Reference In"=w6710, "error in"=w6709, "Scan steps (MCL)"="Scan steps (MCL)", "Number of scans (MCL)"=w6679, "Cycles per step (MCL)"=w6697, "Scan freq.  increment (MCL)"=w6677, "1D or 2D Scan?"="2D or 1D Scan", "MCL Scan Axis"=w6684, "Cont. Scan (MCL)"="Continuous MCL Scanning") -> ("error out"=w6708:errorcluster)  [unwired: 1 out]
      }
      event #32 {
        w6847 = 1000.0 ("y")
        n1505 = event-data() -> ()  [unwired: 7 out]
        n1506 = local read "Save file name"() -> (w6872:path)
        n1507 = local write "Read Cal"(FALSE ("Read Cal")) -> ()
        n1508 = Strip Path(path=w6872) -> (stripped path=w6871:path)  [unwired: 1 out]
        n1509 = Path To String(path=w6871) -> (string=w6870:string)
        n1510 = Concatenate Strings(w6870, "\\current.cal" ("string")) -> (w6868:string)
        n1511 = String To Path(string=w6868) -> (path=w6867:path)
        n1512 = Open/Create/Replace File(file path (use dialog)=w6867, operation (0:open)=T32."open", access (0:read/write)=enum16{"read/write", "read-only", "write-only"}."read-only") -> (refnum out=w6875:refnum<file>, error out=w6861:errorcluster)  [unwired: 1 in, 3 out]
        n1513 = Deny Access(4:w6861, 7:w6875) -> (0:w6860:errorcluster, 3:w6866:refnum<file>)  [unwired: 1 out]
        n1514 = Read from Binary File(5:0.0, 8:w6860, 9:T33."big-endian, network order" ("byte order (0:big-endian, network order)"), 10:-1 ("count (1)"), 11:w6866) -> (0:w6859:errorcluster, 2:w6857:dbl[], 3:w6862:refnum<file>)  [unwired: 2 out]
        n1515 = Array To Cluster(array=w6857) -> (cluster=w6856:T44)
        n1516 = Unbundle(w6856) -> ("[0]"=w6855:dbl, "[1]"=w6854:dbl, "[2]"=w6853:dbl, "[3]"=w6852:dbl, "[4]"=w6851:dbl, "[5]"=w6850:dbl)
        n1517 = Close File(refnum=w6862, error in=w6859) -> (error out=→"Read cal error":errorcluster)  [unwired: 1 out]
        n1518 = Multiply(x=w6850, y=w6847) -> (x*y=w6848:dbl)
        n1519 = local write "T2 kappa_x (pN/nm)"(w6852) -> ()
        n1520 = local write "T1 kappa_x (pN/nm)"(w6853) -> ()
        n1521 = local write "T1 alpha_x (nm/V)"(w6855) -> ()
        n1522 = local write "T2 alpha_x (nm/V)"(w6854) -> ()
        n1523 = Multiply(x=w6851, y=w6847) -> (x*y=w6849:dbl)
        n1524 = local write "T1 offset_x (mV)"(w6849) -> ()
        n1525 = local write "T2 offset_x (mV)"(w6848) -> ()
      }
      event #33 {
        n1526 = event-data() -> ()  [unwired: 7 out]
        n1527 = local write "MCL Scanning"(FALSE ("MCL Scanning")) -> ()
        n1528 = xnode "Read/Write Control"("FPGA VI Reference In"=w6880, "error in"=w6879, "Abort scan (MCL)"="Abort MCL Scan") -> ("error out"=w6878:errorcluster)  [unwired: 1 out]
      }
      event #34 {
        n1529 = event-data() -> ()  [unwired: 7 out]
        n1530 = xnode "Read/Write Control"("FPGA VI Reference In"=w6921, "error in"=w6920, "MCL count"="Update Count (MCL)") -> ("error out"=w6919:errorcluster)  [unwired: 1 out]
      }
      event #35 {
        n1531 = event-data() -> ()  [unwired: 7 out]
        n1532 = Negate(x="Phase adjust (MCL)") -> (-x=w6966:i16)
        n1533 = Select(t=w6966, s="- phase (MCL)", f="Phase adjust (MCL)") -> (s? t:f=w6964:i16)
        n1534 = Or(x="- phase (MCL)", y="+ phase (MCL)") -> (x .or. y?=w6959:bool)
        n1535 = xnode "Read/Write Control"("FPGA VI Reference In"=w6968, "error in"=w6967, "Phase count adjustment (MCL)"=w6964) -> ("FPGA VI Reference Out"=w6960:T20, "error out"=w6961:errorcluster)
        n1536 = xnode "Read/Write Control"("FPGA VI Reference In"=w6960, "error in"=w6961, "+ phase (MCL)"=w6959) -> ("error out"=w6958:errorcluster)  [unwired: 1 out]
      }
      event #36 {
        n1537 = event-data() -> ()  [unwired: 7 out]
        n1538 = xnode "Read/Write Control"("FPGA VI Reference In"=w7045, "error in"=w7044, "Abort scan"="Abort AOD Scan") -> ("error out"=w7043:errorcluster)  [unwired: 1 out]
      }
      event #37 {
        n1539 = event-data() -> ()  [unwired: 7 out]
        n1540 = xnode "Read/Write Control"("FPGA VI Reference In"=w7086, "error in"=w7085, "Cont. Scan"="Continuous AOD Scanning") -> ("error out"=w7084:errorcluster)  [unwired: 1 out]
      }
      event #38 {
        n1541 = event-data() -> ()  [unwired: 7 out]
        n1542 = call "Create new save file.vi"("Insert"="", "Ext"=".dat" ("string"), "Index In"="Index") -> ("Path Out"=→"Save file name":path, "Index Out"=w7124:dbl)
        "Save index" <- w7124
        n1543 = local write "Index"(w7124) -> ()
      }
      event #39 {
        w7139 = 10.0 ("y")
        w7138 = 32767.0 ("y")
        n1544 = event-data() -> ()  [unwired: 7 out]
        n1545 = local read "AO2"() -> (w7137:dbl)
        n1546 = local read "AO1"() -> (w7134:dbl)
        n1547 = Multiply(x=w7134, y=w7138) -> (x*y=w7133:dbl)